vi "Controle_Manip_Main_GUI_Backup2.vi"() -> ()   [LabVIEW 2019] (continued)
                      tunnel: [w4532] -> w4511
                      tunnel: w4510 -> [w4531]
                      tunnel: w4509 -> [w4530]
                      frame #0 {
                        n3649 = call <instrlib>:"TL4000 Get LD Output State.vi"("error in (no error)"=w4516, "instrument handle"=w4523) -> ("error out"=w4518:errorcluster, "LD Output"=w4520:bool, "instrument handle out"=w4519:refnum<visa-resource-name>)  [unwired: 7 in]
                        n3650 = Not(x=w4520) -> (.not. x?=w4517:bool)
                        n3651 = case shown="True" w4517 {
                          selector: w4517 -> [w4525 w4526]
                          frame False {
                            n3652 = Not(x=w4525) -> (.not. x?=w4524:bool)
                            n3653 = property on="TEC Output" class="Bool (strict)"("Visible"=w4524) -> ()  [unwired: 2 in, 2 out]
                          }
                          frame True {
                            n3654 = property on="TEC Output" class="Bool (strict)"("Visible"=w4526) -> ()  [unwired: 2 in, 2 out]
                          }
                        }
                        n3655 = property on="Laser Diode Current Set" class="Slide (strict)"("Visible"=w4517) -> ()  [unwired: 2 in, 2 out]
                        n3656 = property on="Laser Safety" class="Ring (strict)"("Visible"=w4517) -> ()  [unwired: 2 in, 2 out]
                        n3657 = local write "Laser on?"(w4517) -> ()
                        n3658 = call <instrlib>:"TL4000 Switch LD Output.vi"("error in (no error)"=w4518, "LD Output (Off)"=w4517, "instrument handle"=w4519) -> ("error out"=w4522:errorcluster, "instrument handle out"=w4521:refnum<visa-resource-name>)  [unwired: 7 in]
                      }
                      frame #1 {
                        n3659 = local read "PM16-120 On?"() -> (w4527:bool)
                        n3660 = case shown="True" w4527 {
                          tunnel: [w4536 w4543] -> w4533
                          tunnel: [w4537 w4542] -> w4532
                          tunnel: w4531 -> [w4536 w4541]
                          tunnel: w4530 -> [w4537 w4540]
                          tunnel: [0.0 ("Power") w4539] -> w4529
                          frame False {
                          }
                          frame True {
                            n3661 = call <instrlib>:"TLPM Measure Power.vi"("error in (no error)"=w4540, "instrument handle"=w4541) -> ("error out"=w4542:errorcluster, "Power"=w4539:dbl, "instrument handle out"=w4543:refnum<visa-resource-name>)  [unwired: 7 in]
                          }
                        }
                        n3662 = local write "Excitation Power (uW)"(w4529) -> ()
                        n3663 = property on="Excitation Source" class="Enum (strict)"("Val(Sgnl)"=enum16{"P", "CW", "SK"}."CW" ("Value (Signaling)")) -> ()  [unwired: 2 in, 2 out]
                      }
                    }
                  }
                  frame "Laser Diode Current Set" {
                    n3664 = stacked-sequence {
                      seq-local: [w4556 _ _ _] -> [_ _ w4576 _]
                      seq-local: [w4555 _ _ _] -> [_ _ w4575 _]
                      tunnel: w4551 -> [w4560 _ _ _]
                      tunnel: w4544 -> [w4552 _ _ _]
                      tunnel: [_ _ w4576 _] -> w4550
                      tunnel: [_ _ w4575 _] -> w4545
                      tunnel: w4549 -> [_ _ w4574 _]
                      tunnel: w4548 -> [_ _ w4573 _]
                      tunnel: [_ _ w4572 _] -> w4547
                      tunnel: [_ _ w4571 _] -> w4546
                      frame #0 {
                        n3665 = local read "Laser Diode Current Set"() -> (w4553:dbl)
                        n3666 = call <instrlib>:"TL4000 Get Laser Diode Current Setpoint.vi"("error in (no error)"=w4552, "instrument handle"=w4560) -> ("error out"=w4557:errorcluster, "Laser Diode Current Setpoint"=w4559:dbl, "instrument handle out"=w4558:refnum<visa-resource-name>)  [unwired: 7 in]
                        n3667 = Not Equal?(x=w4553, y=w4559) -> (x != y?=w4554:bool)
                        n3668 = case shown="True" w4554 {
                          tunnel: w4558 -> [w4562 w4567]
                          tunnel: w4557 -> [w4561 w4566]
                          tunnel: [w4562 w4565] -> w4556
                          tunnel: [w4561 w4564] -> w4555
                          tunnel: w4553 -> [_ w4563]
                          frame False {
                          }
                          frame True {
                            n3669 = call <instrlib>:"TL4000 Set Laser Diode Current Setpoint.vi"("error in (no error)"=w4566, "Laser Diode Current Setpoint (0.0)"=w4563, "instrument handle"=w4567) -> ("error out"=w4564:errorcluster, "instrument handle out"=w4565:refnum<visa-resource-name>)  [unwired: 7 in]
                          }
                        }
                      }
                      frame #1 {
                        n3670 = Wait (ms)(milliseconds to wait=u32 50) -> ()  [unwired: 1 out]
                      }
                      frame #2 {
                        n3671 = local read "PM16-120 On?"() -> (w4569:bool)
                        n3672 = case shown="True" w4569 {
                          tunnel: w4574 -> [w4579 w4584]
                          tunnel: w4573 -> [w4578 w4583]
                          tunnel: [w4579 w4582] -> w4572
                          tunnel: [w4578 w4581] -> w4571
                          tunnel: [0.0 ("Power") w4580] -> w4570
                          frame False {
                          }
                          frame True {
                            n3673 = call <instrlib>:"TLPM Measure Power.vi"("error in (no error)"=w4583, "instrument handle"=w4584) -> ("error out"=w4581:errorcluster, "Power"=w4580:dbl, "instrument handle out"=w4582:refnum<visa-resource-name>)  [unwired: 7 in]
                          }
                        }
                        n3674 = local write "Excitation Power (uW)"(w4570) -> ()
                      }
                      frame #3 {
                        n3675 = local write "Background taken?"(FALSE ("Background taken?")) -> ()
                      }
                    }
                  }
                  frame "TEC Output" {
                    n3676 = local read "TEC Output"() -> (w4586:bool)
                    n3677 = call <instrlib>:"TL4000 Switch TEC Output.vi"("error in (no error)"=w4587, "TEC Output (Off)"=w4586, "instrument handle"=w4588) -> ("error out"=w4593:errorcluster, "instrument handle out"=w4594:refnum<visa-resource-name>)  [unwired: 7 in]
                    n3678 = case shown="True" w4586 {
                      tunnel: w4594 -> [w4596 w4603]
                      tunnel: w4593 -> [w4595 w4602]
                      tunnel: [w4596 w4599] -> w4590
                      tunnel: [w4595 w4598] -> w4589
                      frame False {
                      }
                      frame True {
                        n3679 = while {
                          tunnel: w4603 -> [w4617]
                          tunnel: [w4609] -> w4600
                          tunnel: w4602 -> [w4616]
                          tunnel: [w4610] -> w4601
                          stop <- w4604 stop-if-true
                          n3680 = call <instrlib>:"TL4000 Measure Temperature.vi"("error in (no error)"=w4616, "instrument handle"=w4617) -> ("error out"=w4610:errorcluster, "Temperature"=w4607:dbl, "instrument handle out"=w4609:refnum<visa-resource-name>)  [unwired: 7 in]
                          n3681 = Wait (ms)(milliseconds to wait=u32 250) -> ()  [unwired: 1 out]
                          n3682 = local write "TEC Temperature"(w4607) -> ()
                          n3683 = Subtract(x=w4607, y=25.0) -> (x-y=w4614:dbl)
                          n3684 = Absolute Value(x=w4614) -> (abs(x)=w4613:dbl)
                          n3685 = Equal?(x=w4607, y=0.0) -> (x = y?=w4605:bool)
                          n3686 = Less?(x=w4613, y=0.01) -> (x < y?=w4608:bool)
                          n3687 = Or(x=w4608, y=w4605) -> (x .or. y?=w4604:bool)
                        }
                        n3688 = call <instrlib>:"TL4000 Measure Temperature.vi"("error in (no error)"=w4601, "instrument handle"=w4600) -> ("error out"=w4598:errorcluster, "Temperature"=w4597:dbl, "instrument handle out"=w4599:refnum<visa-resource-name>)  [unwired: 7 in]
                        n3689 = local write "TEC Temperature"(w4597) -> ()
                      }
                    }
                    n3690 = property on="Laser on? Control" class="Bool (strict)"("Visible"=w4586) -> ()  [unwired: 2 in, 2 out]
                  }
                  frame Default {
                  }
                }
                "Diode Driver Error out" <- w4492
                n3691 = local write "Photodiode error out"(w4490) -> ()
                n3692 = local write "Photodiode handle out"(w4495) -> ()
                n3693 = local write "Diode Driver COM"(w4494) -> ()
              }
            }
          }
          event "Fit?": Mouse Down {
            n3694 = event-data() -> ()  [unwired: 1 in, 8 out]
            n3695 = property on="CCD 1D Spectrum Main" class="XYGraph (strict)"() -> ("Value"=w4626:cluster{dbl[], dbl[]})  [unwired: 2 in, 2 out]
            n3696 = local read "BackgroundSpec"() -> (w4622:dbl[])
            n3697 = Unbundle(w4626) -> (w4625:dbl[], w4623:dbl[])
            n3698 = call "subVI_FitLorentzien.vi"("Background Spec"=w4622, "X"=w4625, "Y"=w4623) -> ("best fit parameters"=→"best fit parameters":dbl[])  [unwired: 1 in, 3 out]
          }
          event "Temperature (K)": Mouse Down {
            n3699 = event-data() -> ()  [unwired: 1 in, 8 out]
            n3700 = local read "Cryostation On?"() -> (w4627:bool)
            n3701 = case shown="True" w4627 {
              frame False {
              }
              frame True {
                w4629 = 10.0 ("y")
                n3702 = local read "Cryostation ID"() -> (w4639:refnum<k5>)
                n3703 = call "GetCryoInfo.vi"("connection ID"=w4639) -> ("User Stability"=w4634:dbl, "User Temp"=w4635:dbl, "connection ID out"=w4633:refnum<k5>, "Sample Stability"=w4636:dbl, "Sample Temp"=w4632:dbl, "Platform Stability"=w4637:dbl, "Platform Temp"=w4638:dbl)  [unwired: 4 in]
                n3704 = local write "Cryo Platform Temp"(w4638) -> ()
                n3705 = Multiply(x=w4632, y=w4629) -> (x*y=w4631:dbl)
                n3706 = local write "Cryo Sample Stability"(w4636) -> ()
                n3707 = local write "Cryostation ID"(w4633) -> ()
                n3708 = local write "Cryo User Stability"(w4634) -> ()
                n3709 = local write "Cryo Sample Temp"(w4632) -> ()
                n3710 = local write "Cryo Platform Stability"(w4637) -> ()
                n3711 = local write "Cryo User Temp"(w4635) -> ()
                n3712 = Round To Nearest(number=w4631) -> (nearest integer value=w4630:dbl)
                n3713 = Divide(x=w4630, y=w4629) -> (x/y=w4628:dbl)
                n3714 = local write "Temperature (K)"(w4628) -> ()
              }
            }
          }
          event "Voltage Output?": Value Change {
            w4644 = u8 2 items=["1", "2", "3"] ("axis")
            w4645 = u8 1 items=["1", "2", "3"] ("axis")
            w4646 = u8 0 items=["1", "2", "3"] ("axis")
            n3715 = event-data() -> ("NewVal"=w4640:bool)  [unwired: 1 in, 5 out]
            n3716 = local read "Att Error"() -> (w4653:errorcluster)
            n3717 = local read "Att DeviceHandle"() -> (w4655:u64)
            n3718 = local read "ourDLL"() -> (w4643:path)
            n3719 = call "ANC350v4_SetAxisOutput.vi"("deviceHandle"=w4655, "Path to *.DLL"=w4643, "axis"=w4646, "enable"=w4640, "autoDisable"=TRUE, "error in"=w4653) -> ("deviceHandle"=w4651:u64, "error ANC350v4_setAxisOutput"=w4652:errorcluster)  [unwired: 7 in, 1 out]
            n3720 = call "ANC350v4_SetAxisOutput.vi"("deviceHandle"=w4651, "Path to *.DLL"=w4643, "axis"=w4645, "enable"=w4640, "autoDisable"=TRUE, "error in"=w4652) -> ("deviceHandle"=w4650:u64, "error ANC350v4_setAxisOutput"=w4649:errorcluster)  [unwired: 7 in, 1 out]
            n3721 = call "ANC350v4_SetAxisOutput.vi"("deviceHandle"=w4650, "Path to *.DLL"=w4643, "axis"=w4644, "enable"=w4640, "autoDisable"=TRUE, "error in"=w4649) -> ("deviceHandle"=w4642:u64, "error ANC350v4_setAxisOutput"=w4641:errorcluster)  [unwired: 7 in, 1 out]
            n3722 = local write "Att Error"(w4641) -> ()
            n3723 = local write "Att DeviceHandle"(w4642) -> ()
          }
          event Timeout {
            # "Use timeout case to send data to globals"
            n3724 = event-data() -> ()  [unwired: 1 in, 3 out]
          }
        }
      }
      n3725 = while {
        stop <- w723 stop-if-true
        # "Separate loop for \"measurements\" requiring simultaneous optimisation of experimental parameters"
        n3726 = event shown="[2] \"Acquire PD\": Mouse Down" {
          selector: _ -> [_ _ _]
          dyn-events: _ -> [_ _ _]
          timeout: 500 -> [_ _ _]
          event Timeout {
            n3727 = event-data() -> ()  [unwired: 1 in, 3 out]
          }
          event "Fast Acq Continuous": Mouse Down {
            n3728 = event-data() -> ()  [unwired: 1 in, 8 out]
            n3729 = local read "Acq Mode"() -> (w724:T3)
            n3730 = case shown="\"Spectrum\", Default" w724 {
              frame "Image" {
              }
              frame "APD 1" {
              }
              frame "Spectrum", Default {
                n3731 = stacked-sequence {
                  frame #0 {
                    # "prep stuff"
                    n3732 = property on="Experiment Graph Controls" class="TabCtl (strict)"("Value"=T25."Spectrum" ("Experiment Graph Controls")) -> ()  [unwired: 2 in, 2 out]
                  }
                  frame #1 {
                    # "open shutter once"
                    n3733 = control-ref of="Shutter Ctrls"() -> (w731:refnum<vi>)
                    n3734 = local read "KCube Shutter On?"() -> (w728:bool)
                    n3735 = local read "Acq Mode"() -> (w729:T3)
                    n3736 = control-ref of="KCube Shutter Device Reference"() -> (w730:refnum<vi>)
                    n3737 = call "Shutter.vi"("KCube Shutter Device Reference 2"=w730, "Shutter Ctrls 2"=w731, "Shutter on?"=w728) -> ()
                    n3738 = case shown="\"Spectrum\", Default" w729 {
                      frame "Spectrum", Default {
                        n3739 = property on="CCD 1D Spectrum Main" class="XYGraph (strict)"("Visible"=TRUE) -> ()  [unwired: 2 in, 2 out]
                        n3740 = property on="CCD 2D Image Main" class="IntGraph (strict)"("Visible"=FALSE) -> ()  [unwired: 2 in, 2 out]
                      }
                      frame "Image" {
                        n3741 = property on="CCD 1D Spectrum Main" class="XYGraph (strict)"("Visible"=FALSE) -> ()  [unwired: 2 in, 2 out]
                        n3742 = property on="CCD 2D Image Main" class="IntGraph (strict)"("Visible"=TRUE) -> ()  [unwired: 2 in, 2 out]
                      }
                    }
                    n3743 = control-ref of="MasterStop"() -> (w727:refnum<vi>)
                    n3744 = property class="Bool (strict)"(reference=w727, "Visible"=TRUE) -> ()  [unwired: 1 in, 2 out]
                  }
                  frame #2 {
                    # "acquire 1000 spectra"
                    n3745 = for {
                      N: 1000 -> [_]
                      stop <- w751 stop-if-true
                      n3746 = local read "CCD ROI"() -> (w746:T20)
                      n3747 = local read "LightField Automation out"() -> (w750:refnum<class "LightField Automation.lvclass">)
                      n3748 = local read "Acq Mode"() -> (w753:T3)
                      n3749 = local read "LightField Automation error out"() -> (w747:errorcluster)
                      n3750 = local read "Accumulations"() -> (w754:dbl)
                      n3751 = control-ref of="MasterStop"() -> (w737:refnum<vi>)
                      n3752 = local read "BackgroundSpec"() -> (w739:dbl[])
                      n3753 = local read "Excitation Power (uW)"() -> (w742:dbl)
                      n3754 = call "LFA_Capture.vi"("error in (no error)"=w747, "Frames"=w754, "LightField Automation in"=w750) -> ("error out"=w748:errorcluster, "Data"=w752:T26, "LightField Automation out"=w749:refnum<class "LightField Automation.lvclass">)  [unwired: 6 in]
                      n3755 = case shown="\"Spectrum\", Default" w753 {
                        selector: w753 -> [w762 w768]
                        tunnel: w752 -> [w763 w770]
                        tunnel: w746 -> [w759 w765]
                        tunnel: [w755 w764] -> w743
                        frame "Spectrum", Default {
                          n3756 = local read "Wavelength calibration"() -> (w757:dbl[])
                          n3757 = Divide(x=1239.842, y=w757) -> (x/y=w756:dbl[])
                          n3758 = call "PrepareData4Graph.vi"("Wavelength nm"=w756, "DataLF"=w763, "CCD ROI"=w759, "AcqMode"=w762, "Data type"=T30."Spectre") -> ("Spectrum"=w761:cluster{"Array 2":dbl[], "Array":dbl[]}, "PLInt out"=w755:dbl[])  [unwired: 2 in, 2 out]
                          n3759 = local write "CCD 1D Spectrum Main"(w761) -> ()
                        }
                        frame "Image" {
                          n3760 = local read "Wavelength calibration"() -> (w769:dbl[])
                          n3761 = call "PrepareData4Graph.vi"("Wavelength nm"=w769, "DataLF"=w770, "CCD ROI"=w765, "AcqMode"=w768, "Data type"=T30."Spectre") -> ("Intensity Graph"=w767:dbl[][], "PLInt out"=w764:dbl[])  [unwired: 2 in, 2 out]
                          n3762 = local write "CCD 2D Image Main"(w767) -> ()
                        }
                      }
                      n3763 = call "myMax.vi"("Array"=w743) -> ("myMax"=w745:dbl)  [unwired: 1 in]
                      n3764 = property on="CCD 1D Spectrum Main" class="XYGraph (strict)"("YScale.Maximum"=w745, "YScale.Minimum"=0.0 ("Y Scale.Range:Minimum")) -> ()  [unwired: 2 in, 2 out]
                      n3765 = local read "Acq Time (ms)"() -> (w741:dbl)
                      n3766 = local read "Display Mode"() -> (w738:u16)
                      n3767 = local write "LightField Automation out"(w749) -> ()
                      n3768 = local write "LightField Automation error out"(w748) -> ()
                      n3769 = property class="Bool (strict)"(reference=w737) -> ("Value"=w751:bool)  [unwired: 1 in, 2 out]
                      n3770 = control-ref of="Cnts"() -> (w740:refnum<vi>)
                      n3771 = call "2Cnts.vi"("Array Background"=w739, "Pow W"=w742, "AcqTime ms"=w741, "Cnts Ref"=w740, "Display Mode"=w738, "Array"=w743) -> ()  [unwired: 1 out]
                    }
                  }
                  frame #3 {
                    # "close shutter"
                    n3772 = local read "KCube Shutter On?"() -> (w774:bool)
                    n3773 = control-ref of="Fast Acq Continuous"() -> (w772:refnum<vi>)
                    n3774 = control-ref of="Shutter Ctrls"() -> (w778:refnum<vi>)
                    n3775 = control-ref of="KCube Shutter Device Reference"() -> (w777:refnum<vi>)
                    n3776 = control-ref of="MasterStop"() -> (w773:refnum<vi>)
                    n3777 = property class="Bool (strict)"(reference=w772, "Value"=FALSE) -> ()  [unwired: 1 in, 2 out]
                    n3778 = call "Shutter.vi"("KCube Shutter Device Reference 2"=w777, "Shutter Ctrls 2"=w778, "Shutter on?"=w774) -> ()
                    n3779 = property class="Bool (strict)"(reference=w773, "Value"=FALSE, "Visible"=FALSE) -> ()  [unwired: 1 in, 2 out]
                  }
                }
              }
            }
          }
          event "Acquire PD": Mouse Down {
            n3780 = event-data() -> ()  [unwired: 1 in, 8 out]
            n3781 = local read "PicoHarp On?"() -> (w779:bool)
            n3782 = case shown="True" w779 {
              frame False {
              }
              frame True {
                n3783 = local read "Spectrum Custom Continuous Mode"() -> (w780:u16)
                n3784 = case shown="3" w780 {
                  frame 0, Default {
                    # "PD 2"
                    n3785 = stacked-sequence {
                      frame #0 {
                        n3786 = property on="Experiment Graph Controls" class="TabCtl (strict)"("Value"=T25."APDs" ("Experiment Graph Controls")) -> ()  [unwired: 2 in, 2 out]
                      }
                      frame #1 {
                        n3787 = for {
                          N: 1000 -> [_]
                          shift-right: [w786] -> _
                          shift-left: dbl[] [] -> [w791]
                          stop <- w784 stop-if-true
                          n3788 = local read "Photodiode handle out"() -> (w797:refnum<visa-resource-name>)
                          n3789 = local read "Photodiode error out"() -> (w796:errorcluster)
                          n3790 = control-ref of="PD 1D Spectrum"() -> (w788:refnum<vi>)
                          n3791 = Tick Count (ms)() -> (millisecond timer value=w793:u32)
                          n3792 = while {
                            shift-right: [w807] -> w795
                            shift-left: w797 -> [w810]
                            shift-right: [w806] -> w794
                            shift-left: w796 -> [w809]
                            tunnel: w793 -> [w803]
                            shift-right: [w798] -> w790
                            shift-left: dbl[] [] -> [w800]
                            stop <- w802 stop-if-true
                            n3793 = local read "Acq Time (ms)"() -> (w801:dbl)
                            n3794 = Tick Count (ms)() -> (millisecond timer value=w805:u32)
                            n3795 = call <instrlib>:"TLPM Measure Power.vi"("error in (no error)"=w809, "instrument handle"=w810) -> ("error out"=w806:errorcluster, "Power"=w799:dbl, "instrument handle out"=w807:refnum<visa-resource-name>)  [unwired: 7 in]
                            n3796 = control-ref of="Excitation Power (uW)"() -> (w808:refnum<vi>)
                            n3797 = property class="DigNum (strict)"(reference=w808, "Value"=w799) -> ()  [unwired: 1 in, 2 out]
                            n3798 = Subtract(x=w805, y=w803) -> (x-y=w804:u32)
                            n3799 = Insert Into Array(array=w800, new element=w799) -> (w798:dbl[])  [unwired: 1 in]
                            n3800 = Greater?(x=w804, y=w801) -> (0:w802:bool)
                          }
                          n3801 = control-ref of="Stop PD"() -> (w785:refnum<vi>)
                          n3802 = local write "Photodiode handle out"(w795) -> ()
                          n3803 = call-poly <vilib>:"Mean.vi"("X"=w790) -> ("mean"=w789:dbl)  [unwired: 1 out]
                          n3804 = Insert Into Array(array=w791, new element=w789) -> (w786:dbl[])  [unwired: 1 in]
                          n3805 = Build Array(w786) -> (w787:dbl[][])
                          n3806 = property class="WFGraph (strict)"(reference=w788, "Value"=w787) -> ()  [unwired: 1 in, 2 out]
                          n3807 = local write "Photodiode error out"(w794) -> ()
                          n3808 = property class="Bool (strict)"(reference=w785) -> ("Value"=w784:bool)  [unwired: 1 in, 2 out]
                        }
                      }
                      frame #2 {
                        w811 = FALSE ("Stop PD")
                        n3809 = property on="Acquire PD" class="Bool (strict)"("Value"=w811) -> ()  [unwired: 2 in, 2 out]
                        n3810 = property on="Stop PD" class="Bool (strict)"("Value"=w811) -> ()  [unwired: 2 in, 2 out]
                      }
                    }
                  }
                  frame 3 {
                    # "APD1+2"
                    n3811 = stacked-sequence {
                      frame #0 {
                        n3812 = local read "PH_Init_Data"() -> (w824:T11)
                        n3813 = Unbundle By Name(w824) -> ("Deviceindex"=w816:i32)
                        n3814 = local read "PH_Settings_Params"() -> (w817:T10)
                        n3815 = local read "PH_CFD1 level"() -> (w821:i32)
                        n3816 = local read "PH_CFD1 zero X"() -> (w820:i32)
                        n3817 = local read "Acq Time (ms)"() -> (w819:dbl)
                        n3818 = local read "PH_Range No."() -> (w815:i32)
                        n3819 = local read "PH_CFD0 level"() -> (w822:i32)
                        n3820 = local read "PH_CFD0 zero X"() -> (w814:i32)
                        n3821 = local read "PH_SyncDiv"() -> (w823:enum16{"1", "2", "4", "8"})
                        n3822 = property on="Experiment Graph Controls" class="TabCtl (strict)"("Value"=T25."APDs" ("Experiment Graph Controls")) -> ()  [unwired: 2 in, 2 out]
                        n3823 = Bundle By Name(cluster=w817, "SyncDiv"=w823, "DeviceIndex"=w816, "CFD0 level"=w822, "CFD0 zero X"=w814, "CFD1 level"=w821, "CFD1 zero X"=w820, "Range No."=w815, "StopOnOverflow"=TRUE, "AcqTime (ms)"=w819) -> (w812:T10)
                        n3824 = local write "PH_Settings_Params"(w812) -> ()
                      }
                      frame #1 {
                        n3825 = local read "PH_Init_Data"() -> (w827:T11)
                        n3826 = local read "PH_Settings_Params"() -> (w828:T10)
                        n3827 = control-ref of="Stop PD"() -> (w829:refnum<vi>)
                        n3828 = control-ref of="PD 1D Spectrum"() -> (w830:refnum<vi>)
                        n3829 = call "PH_GetRates_SubVI.vi"("APD num"=enum16{"NA", "APD1", "APD2", "APD1+2"}."APD1+2", "PH_Settings_Params"=w828, "PH_Init_Data"=w827, "Stop PD Ref"=w829, "PD 1D Spectrum Ref"=w830) -> ("APD1+2"=w825:dbl[][])  [unwired: 6 in]
                        n3830 = local write "PD Data 2D 2"(w825) -> ()
                      }
                      frame #2 {
                        w831 = FALSE ("Stop PD")
                        n3831 = property on="Acquire PD" class="Bool (strict)"("Value"=w831) -> ()  [unwired: 2 in, 2 out]
                        n3832 = property on="Stop PD" class="Bool (strict)"("Value"=w831) -> ()  [unwired: 2 in, 2 out]
                      }
                    }
                  }
                  frame 1 {
                    # "APD1"
                    n3833 = stacked-sequence {
                      frame #0 {
                        n3834 = local read "PH_Init_Data"() -> (w844:T11)
                        n3835 = Unbundle By Name(w844) -> ("Deviceindex"=w836:i32)
                        n3836 = local read "PH_Settings_Params"() -> (w837:T10)
                        n3837 = local read "PH_CFD1 level"() -> (w841:i32)
                        n3838 = local read "PH_CFD1 zero X"() -> (w840:i32)
                        n3839 = local read "Acq Time (ms)"() -> (w839:dbl)
                        n3840 = local read "PH_Range No."() -> (w835:i32)
                        n3841 = local read "PH_CFD0 level"() -> (w842:i32)
                        n3842 = local read "PH_CFD0 zero X"() -> (w834:i32)
                        n3843 = local read "PH_SyncDiv"() -> (w843:enum16{"1", "2", "4", "8"})
                        n3844 = property on="Experiment Graph Controls" class="TabCtl (strict)"("Value"=T25."APDs" ("Experiment Graph Controls")) -> ()  [unwired: 2 in, 2 out]
                        n3845 = Bundle By Name(cluster=w837, "SyncDiv"=w843, "DeviceIndex"=w836, "CFD0 level"=w842, "CFD0 zero X"=w834, "CFD1 level"=w841, "CFD1 zero X"=w840, "Range No."=w835, "StopOnOverflow"=TRUE, "AcqTime (ms)"=w839) -> (w832:T10)
                        n3846 = local write "PH_Settings_Params"(w832) -> ()
                      }
                      frame #1 {
                        n3847 = local read "PH_Init_Data"() -> (w847:T11)
                        n3848 = local read "PH_Settings_Params"() -> (w848:T10)
                        n3849 = control-ref of="Stop PD"() -> (w849:refnum<vi>)
                        n3850 = control-ref of="PD 1D Spectrum"() -> (w850:refnum<vi>)
                        n3851 = call "PH_GetRates_SubVI.vi"("APD num"=enum16{"NA", "APD1", "APD2", "APD1+2"}."APD1", "PH_Settings_Params"=w848, "PH_Init_Data"=w847, "Stop PD Ref"=w849, "PD 1D Spectrum Ref"=w850) -> ("APD1+2"=w845:dbl[][])  [unwired: 6 in]
                        n3852 = local write "PD Data 2D 2"(w845) -> ()
                      }
                      frame #2 {
                        w851 = FALSE ("Stop PD")
                        n3853 = property on="Acquire PD" class="Bool (strict)"("Value"=w851) -> ()  [unwired: 2 in, 2 out]
                        n3854 = property on="Stop PD" class="Bool (strict)"("Value"=w851) -> ()  [unwired: 2 in, 2 out]
                      }
                    }
                  }
                  frame 2 {
                    # "APD2"
                    n3855 = stacked-sequence {
                      frame #0 {
                        n3856 = local read "PH_Init_Data"() -> (w864:T11)
                        n3857 = Unbundle By Name(w864) -> ("Deviceindex"=w856:i32)
                        n3858 = local read "PH_Settings_Params"() -> (w857:T10)
                        n3859 = local read "PH_CFD1 level"() -> (w861:i32)
                        n3860 = local read "PH_CFD1 zero X"() -> (w860:i32)
                        n3861 = local read "Acq Time (ms)"() -> (w859:dbl)
                        n3862 = local read "PH_Range No."() -> (w855:i32)
                        n3863 = local read "PH_CFD0 level"() -> (w862:i32)
                        n3864 = local read "PH_CFD0 zero X"() -> (w854:i32)
                        n3865 = local read "PH_SyncDiv"() -> (w863:enum16{"1", "2", "4", "8"})
                        n3866 = property on="Experiment Graph Controls" class="TabCtl (strict)"("Value"=T25."APDs" ("Experiment Graph Controls")) -> ()  [unwired: 2 in, 2 out]
                        n3867 = Bundle By Name(cluster=w857, "SyncDiv"=w863, "DeviceIndex"=w856, "CFD0 level"=w862, "CFD0 zero X"=w854, "CFD1 level"=w861, "CFD1 zero X"=w860, "Range No."=w855, "StopOnOverflow"=TRUE, "AcqTime (ms)"=w859) -> (w852:T10)
                        n3868 = local write "PH_Settings_Params"(w852) -> ()
                      }
                      frame #1 {
                        n3869 = local read "PH_Init_Data"() -> (w867:T11)
                        n3870 = local read "PH_Settings_Params"() -> (w868:T10)
                        n3871 = control-ref of="Stop PD"() -> (w869:refnum<vi>)
                        n3872 = control-ref of="PD 1D Spectrum"() -> (w870:refnum<vi>)
                        n3873 = call "PH_GetRates_SubVI.vi"("APD num"=enum16{"NA", "APD1", "APD2", "APD1+2"}."APD2", "PH_Settings_Params"=w868, "PH_Init_Data"=w867, "Stop PD Ref"=w869, "PD 1D Spectrum Ref"=w870) -> ("APD1+2"=w865:dbl[][])  [unwired: 6 in]
                        n3874 = local write "PD Data 2D 2"(w865) -> ()
                      }
                      frame #2 {
                        w871 = FALSE ("Stop PD")
                        n3875 = property on="Acquire PD" class="Bool (strict)"("Value"=w871) -> ()  [unwired: 2 in, 2 out]
                        n3876 = property on="Stop PD" class="Bool (strict)"("Value"=w871) -> ()  [unwired: 2 in, 2 out]
                      }
                    }
                  }
                }
              }
            }
          }
        }
        n3877 = local read "NewVal"() -> (w723:bool)
      }
    }
    frame #3 {
      # "Shutdown: close all open references and connections"
      n3878 = stacked-sequence {
        frame #0 {
          # "Is the sample to be kept and reused?\ni.e. does LabVIEW keep sample details or empty them"
          n3879 = Two Button Dialog(message="Do you want to keep the sample details in LV?", 1:"No thanks." ("F button name (\"Cancel\")"), 2:"Yes please!" ("T button name (\"OK\")")) -> (T button?=w4656:bool)
          n3880 = case shown="False" w4656 {
            frame False {
              n3881 = local write "SampleGoal"("") -> ()
            }
            frame True {
            }
          }
        }
        frame #1 {
          # "Shutdown all connections"
          n3882 = local read "Initialise all devices?"() -> (w4661:bool)
          n3883 = case shown="True" w4661 {
            frame False {
              # "No devices to deactivate"
            }
            frame True {
              # "Deactivate all the selected devices"
              n3884 = stacked-sequence {
                frame #0 {
                  # "Message to user"
                  n3885 = local read "Log file"() -> (w4665:string)
                  n3886 = call "Write2LogFile.vi"("Add to log file"="Closing all connections ...", "Log file before"=w4665, "Checkbox"=FALSE) -> ("Log file after"=w4664:string)
                  n3887 = local write "Log file"(w4664) -> ()
                }
                frame #1 {
                  # "LLTF"
                  n3888 = local read "LLTF On?"() -> (w4666:bool)
                  n3889 = case shown="True" w4666 {
                    frame False {
                    }
                    frame True {
                      n3890 = local read "LLTF Reference"() -> (w4668:refnum<k7>)
                      n3891 = local read "LLTF Error"() -> (w4667:errorcluster)
                      n3892 = Close Reference(reference=w4668, error in (no error)=w4667) -> ()  [unwired: 1 out]
                    }
                  }
                }
                frame #2 {
                  # "turn off laser output, TEC and close connection"
                  # "448.3nm Laser Diode + Temp Controller & Driver"
                  n3893 = local read "Laser Comm On?"() -> (w4669:bool)
                  n3894 = case shown="True" w4669 {
                    frame False {
                      w4670 = TRUE ("Visible")
                      n3895 = property on="TEC Output" class="Bool (strict)"("Visible"=w4670) -> ()  [unwired: 2 in, 2 out]
                      n3896 = property on="TEC Temperature" class="DigNum (strict)"("Visible"=w4670) -> ()  [unwired: 2 in, 2 out]
                    }
                    frame True {
                      w4672 = FALSE ("TEC Output (Off)")
                      w4671 = FALSE ("LD Output (Off)")
                      # "laser"
                      n3897 = local read "Diode Driver COM"() -> (w4674:refnum<visa-resource-name>)
                      n3898 = local read "Diode Driver Error"() -> (w4673:errorcluster)
                      n3899 = property on="Laser on? Control" class="Bool (strict)"("Visible"=w4671) -> ()  [unwired: 2 in, 2 out]
                      n3900 = Not(x=w4671) -> (.not. x?=w4679:bool)
                      n3901 = call <instrlib>:"TL4000 Switch LD Output.vi"("error in (no error)"=w4673, "LD Output (Off)"=w4671, "instrument handle"=w4674) -> ("error out"=w4675:errorcluster, "instrument handle out"=w4678:refnum<visa-resource-name>)  [unwired: 7 in]
                      n3902 = property on="Laser Safety" class="Ring (strict)"("Visible"=w4671) -> ()  [unwired: 2 in, 2 out]
                      n3903 = local write "Laser on?"(w4671) -> ()
                      n3904 = local write "Laser on? Control"(w4671) -> ()
                      n3905 = property on="TEC Output" class="Bool (strict)"("Visible"=w4679) -> ()  [unwired: 2 in, 2 out]
                      n3906 = call <instrlib>:"TL4000 Switch TEC Output.vi"("error in (no error)"=w4675, "TEC Output (Off)"=w4672, "instrument handle"=w4678) -> ("error out"=w4676:errorcluster, "instrument handle out"=w4677:refnum<visa-resource-name>)  [unwired: 7 in]
                      n3907 = call <instrlib>:"TL4000 Close.vi"("error in (no error)"=w4676, "instrument handle"=w4677) -> ()  [unwired: 9 in, 1 out]
                      n3908 = local write "TEC Output"(w4672) -> ()
                      n3909 = property on="Laser Diode Current Set" class="Slide (strict)"("Visible"=w4671) -> ()  [unwired: 2 in, 2 out]
                      n3910 = property on="TEC Temperature" class="DigNum (strict)"("Visible"=w4679) -> ()  [unwired: 2 in, 2 out]
                    }
                  }
                }
                frame #3 {
                  # "KCubes: 1 Shutter + 3 Piezos"
                  n3911 = local read "KCubes Piezo On?"() -> (w4681:bool)
                  n3912 = case shown="True" w4681 {
                    frame False {
                    }
                    frame True {
                      # "Close piezo controls and shutter device"
                      n3913 = local read "KCubePiezoControl Y Reference"() -> (w4684:refnum<k24>)
                      n3914 = local read "KCubePiezoControl X Reference"() -> (w4683:refnum<k24>)
                      n3915 = local read "KCubePiezoControl Z Reference"() -> (w4685:refnum<k24>)
                      n3916 = invoke class="KCubePiezoControl" method="CloseDevice"(reference=w4684) -> ()  [unwired: 2 in, 3 out]
                      n3917 = invoke class="KCubePiezoControl" method="CloseDevice"(reference=w4683) -> ()  [unwired: 2 in, 3 out]
                      n3918 = invoke class="KCubePiezoControl" method="CloseDevice"(reference=w4685) -> ()  [unwired: 2 in, 3 out]
                    }
                  }
                  n3919 = local read "KCube Shutter On?"() -> (w4680:bool)
                  n3920 = case shown="True" w4680 {
                    frame False {
                    }
                    frame True {
                      n3921 = local read "KCubeSolenoidControl Reference"() -> (w4682:refnum<k24>)
                      n3922 = invoke class="KCubeSolenoidControl" method="CloseDevice"(reference=w4682) -> ()  [unwired: 2 in, 3 out]
                    }
                  }
                }
                frame #4 {
                  # "LightField: SpectraPro Mono + CCD"
                  n3923 = local read "LightField On?"() -> (w4686:bool)
                  n3924 = case shown="True" w4686 {
                    frame False {
                    }
                    frame True {
                      n3925 = local read "LightField Automation error out"() -> (w4687:errorcluster)
                      n3926 = local read "LightField Automation out"() -> (w4688:refnum<class "LightField Automation.lvclass">)
                      n3927 = call "LFA_Close.vi"("error in (no error)"=w4687, "LightField Automation in"=w4688) -> ()  [unwired: 8 in, 2 out]
                    }
                  }
                }
                frame #5 {
                  # "ESP 301: 2 rotation stages + 1 linear translation stage"
                  n3928 = local read "ESP 301 On?"() -> (w4689:bool)
                  n3929 = case shown="True" w4689 {
                    frame False {
                    }
                    frame True {
                      n3930 = local read "ESP 301 COM Port"() -> (w4690:refnum<visa-resource-name>)
                      n3931 = call "Close.vi"("VISA resource name"=w4690) -> ()  [unwired: 10 in, 1 out]
                    }
                  }
                }
                frame #6 {
                  # "ESP 300: Mono Jobin Yvon"
                  n3932 = local read "ESP 300 On?"() -> (w4691:bool)
                  n3933 = case shown="True" w4691 {
                    frame False {
                    }
                    frame True {
                      n3934 = local read "ESP300 COM Port"() -> (w4692:refnum<visa-resource-name>)
                      n3935 = local read "ESP300 Error"() -> (w4693:errorcluster)
                      n3936 = call "Uninit Communication.vi"("error in (no error)"=w4693, "VISA resource name in"=w4692) -> ()  [unwired: 9 in, 1 out]
                    }
                  }
                }
                frame #7 {
                  # "Thorlabs USB photodiode"
                  n3937 = local read "PM16-120 On?"() -> (w4694:bool)
                  n3938 = case shown="True" w4694 {
                    frame False {
                    }
                    frame True {
                      # "photo"
                      n3939 = local read "Photodiode error out"() -> (w4699:errorcluster)
                      n3940 = call <instrlib>:"TLPM Measure Power.vi"("error in (no error)"=w4699, "instrument handle"=refnum<visa-resource-name> "USB0::0x1313::0x807B::190927109::INSTR") -> ("error out"=w4697:errorcluster, "Power"=w4696:dbl, "instrument handle out"=w4698:refnum<visa-resource-name>)  [unwired: 7 in]
                      n3941 = call <instrlib>:"TLPM Close.vi"("error in (no error)"=w4697, "instrument handle"=w4698) -> ("error out"=w4700:errorcluster)  [unwired: 9 in]
                      n3942 = local write "Excitation Power (uW)"(w4696) -> ()
                      n3943 = local write "Photodiode error out"(w4700) -> ()
                    }
                  }
                }
                frame #8 {
                  # "Attocubes disconnect"
                  n3944 = local read "Attocubes On?"() -> (w4701:bool)
                  n3945 = case shown="True" w4701 {
                    frame False {
                    }
                    frame True {
                      w4707 = u8 2 items=["1", "2", "3"] ("axis")
                      w4708 = u8 1 items=["1", "2", "3"] ("axis")
                      w4717 = u8 0 items=["1", "2", "3"] ("axis")
                      w4706 = FALSE ("ANC connected")
                      n3946 = local read "Att DeviceHandle"() -> (w4719:u64)
                      n3947 = local read "Att Error"() -> (w4718:errorcluster)
                      n3948 = local read "ourDLL"() -> (w4705:path)
                      n3949 = call "ANC350v4_SetAxisOutput.vi"("deviceHandle"=w4719, "Path to *.DLL"=w4705, "axis"=w4717, "enable"=FALSE, "autoDisable"=TRUE, "error in"=w4718) -> ("deviceHandle"=w4711:u64, "error ANC350v4_setAxisOutput"=w4716:errorcluster)  [unwired: 7 in, 1 out]
                      n3950 = call "ANC350v4_SetAxisOutput.vi"("deviceHandle"=w4711, "Path to *.DLL"=w4705, "axis"=w4708, "enable"=FALSE, "autoDisable"=TRUE, "error in"=w4716) -> ("deviceHandle"=w4712:u64, "error ANC350v4_setAxisOutput"=w4715:errorcluster)  [unwired: 7 in, 1 out]
                      n3951 = call "ANC350v4_SetAxisOutput.vi"("deviceHandle"=w4712, "Path to *.DLL"=w4705, "axis"=w4707, "enable"=FALSE, "autoDisable"=TRUE, "error in"=w4715) -> ("deviceHandle"=w4713:u64, "error ANC350v4_setAxisOutput"=w4714:errorcluster)  [unwired: 7 in, 1 out]
                      n3952 = call "ANC350v4sub_Disconnect.vi"("ANC350v4_Handle"=w4713, "Path to *.DLL"=w4705, "error in"=w4714) -> ("error ANC350v4_Dis/Connect"=w4721:errorcluster)  [unwired: 12 in]
                      n3953 = local write "Voltage Output?"(w4706) -> ()
                      n3954 = local write "ANC connected"(w4706) -> ()
                      n3955 = local write "Att Error"(w4721) -> ()
                    }
                  }
                }
                frame #9 {
                  # "Montana Cryostation s50"
                  n3956 = local read "Cryostation On?"() -> (w4722:bool)
                  n3957 = case shown="True" w4722 {
                    frame False {
                    }
                    frame True {
                      n3958 = local read "Cryostation ID"() -> (w4723:refnum<k5>)
                      n3959 = call "CryoDisconnect.vi"("connection ID"=w4723) -> ()
                    }
                  }
                }
                frame #10 {
                  n3960 = local read "PicoHarp On?"() -> (w4724:bool)
                  n3961 = case shown="True" w4724 {
                    frame False {
                    }
                    frame True {
                      n3962 = local read "PH_Init_Data"() -> (w4727:T11)
                      n3963 = Unbundle By Name(w4727) -> ("Deviceindex"=w4726:i32)
                      n3964 = local write "Connected"(FALSE) -> ()
                      n3965 = call "PH_Close.vi"("devidx"=w4726) -> ()
                    }
                  }
                }
              }
            }
          }
        }
        frame #2 {
          # "Save log file & empty strings for next operation"
          n3966 = local read "Initialise all devices?"() -> (w4728:bool)
          n3967 = property on="Experiment Graph Controls" class="TabCtl (strict)"() -> ("Pages"=w4733:refnum<vi>[])  [unwired: 2 in, 2 out]
          n3968 = case shown="True" w4728 {
            frame False {
            }
            frame True {
              n3969 = stacked-sequence {
                frame #0 {
                  # "save log file"
                  n3970 = local read "Experiment Name"() -> (w4736:string)
                  n3971 = local read "Log file"() -> (w4737:string)
                  n3972 = call "CreatePath.vi"("filetype"=enum16{".h5", ".txt"}.".txt", "FileName"=w4736) -> ("File path"=w4734:path)
                  n3973 = Write to Text File(file (use dialog)=w4734, text=w4737) -> ()  [unwired: 2 in, 3 out]
                }
              }
            }
          }
          n3974 = Index Array(array=w4733, index=6) -> (element=w4731:refnum<vi>)
          n3975 = property class="Page"(reference=w4731, "PageVis"=TRUE ("Page Visible")) -> ()  [unwired: 1 in, 2 out]
          n3976 = property on="Experiment Graph Controls" class="TabCtl (strict)"("Value"=T25."Settings" ("Experiment Graph Controls")) -> ()  [unwired: 2 in, 2 out]
        }
      }
    }
  }
  n3977 = disable-structure shown="Disabled" {
    frame Disabled {
      n3978 = stacked-sequence {
        tunnel: [_ _ w4786] -> w4739
        frame #0 {
          n3979 = property on="CCD 1D Spectrum Main" class="XYGraph (strict)"("YScale.Offset"=0.0 ("Y Scale.Offset and Multiplier:Offset")) -> ()  [unwired: 2 in, 2 out]
          n3980 = local read "Log file"() -> (w4771:string)
          n3981 = call "Write2LogFile.vi"("Add to log file"="Acquiring background", "Log file before"=w4771) -> ("Log file after"=w4770:string)
          n3982 = local write "Log file"(w4770) -> ()
        }
        frame #1 {
          # "make sure shutter is closed"
          n3983 = control-ref of="Shutter Ctrls"() -> (w4776:refnum<vi>)
          n3984 = control-ref of="KCube Shutter Device Reference"() -> (w4777:refnum<vi>)
          n3985 = property class="Ring (strict)"(reference=w4776) -> ("Value"=w4775:u16)  [unwired: 1 in, 2 out]
          n3986 = local read "KCube Shutter On?"() -> (w4772:bool)
          n3987 = Equal?(x=w4775, y=u16 0) -> (x = y?=w4773:bool)
          n3988 = case shown="False" w4773 {
            tunnel: w4777 -> [w4780 _]
            tunnel: w4776 -> [w4779 _]
            tunnel: w4772 -> [w4778 _]
            frame False {
              n3989 = call "Shutter.vi"("KCube Shutter Device Reference 2"=w4780, "Shutter Ctrls 2"=w4779, "Shutter on?"=w4778) -> ()
            }
            frame True {
            }
          }
        }
        frame #2 {
          # "acquire"
          n3990 = local read "LightField Automation error out"() -> (w4784:errorcluster)
          n3991 = local read "LightField Automation out"() -> (w4785:refnum<class "LightField Automation.lvclass">)
          n3992 = local read "Accumulations"() -> (w4781:dbl)
          n3993 = call "LFA_Capture.vi"("error in (no error)"=w4784, "Frames"=w4781, "LightField Automation in"=w4785) -> ("error out"=w4783:errorcluster, "Data"=w4786:T26, "LightField Automation out"=w4782:refnum<class "LightField Automation.lvclass">)  [unwired: 6 in]
          n3994 = local write "LightField Automation out"(w4782) -> ()
          n3995 = local write "LightField Automation error out"(w4783) -> ()
        }
      }
      n3996 = local read "Acq Mode"() -> (w4738:T3)
      n3997 = case shown="\"Spectrum\", Default" w4738 {
        selector: w4738 -> [w4740 w4758]
        tunnel: w4739 -> [w4741 w4759]
        frame "Spectrum", Default {
          n3998 = stacked-sequence {
            tunnel: w4741 -> [_ w4752 _ _]
            tunnel: w4740 -> [_ w4750 _ _]
            frame #0 {
              n3999 = property on="CCD 2D Image Main" class="IntGraph (strict)"("Visible"=FALSE) -> ()  [unwired: 2 in, 2 out]
              n4000 = property on="CCD 1D Spectrum Main" class="XYGraph (strict)"("Visible"=TRUE) -> ()  [unwired: 2 in, 2 out]
            }
            frame #1 {
              n4001 = local read "Wavelength calibration"() -> (w4749:dbl[])
              n4002 = local read "CCD ROI"() -> (w4745:T20)
              n4003 = Divide(x=1239.842, y=w4749) -> (x/y=w4747:dbl[])
              n4004 = call "PrepareData4Graph.vi"("Wavelength nm"=w4747, "DataLF"=w4752, "CCD ROI"=w4745, "AcqMode"=w4750, "Data type"=T30."Spectre") -> ("Spectrum"=w4751:cluster{"Array 2":dbl[], "Array":dbl[]}, "PLInt out"=w4744:dbl[])  [unwired: 2 in, 2 out]
              n4005 = local write "CCD 1D Spectrum Main"(w4751) -> ()
              n4006 = local write "BackgroundSpec"(w4744) -> ()
            }
            frame #2 {
              n4007 = local read "BackgroundSpec"() -> (w4753:dbl[])
              n4008 = call-poly <vilib>:"Mean.vi"("X"=w4753) -> ("mean"=w4755:dbl)  [unwired: 1 out]
              n4009 = Negate(x=w4755) -> (-x=w4754:dbl)
              n4010 = property on="CCD 1D Spectrum Main" class="XYGraph (strict)"("YScale.Offset"=w4754) -> ()  [unwired: 2 in, 2 out]
            }
            frame #3 {
              n4011 = local write "Background taken?"(TRUE ("Background taken?")) -> ()
              n4012 = property on="Background substract" class="Enum (strict)"("Value"=enum16{"None", "Shutter"}."None" ("Background substract")) -> ()  [unwired: 2 in, 2 out]
            }
          }
        }
        frame "Image" {
          n4013 = stacked-sequence {
            tunnel: w4759 -> [_ w4767]
            tunnel: w4758 -> [_ w4765]
            frame #0 {
              n4014 = property on="CCD 2D Image Main" class="IntGraph (strict)"("Visible"=TRUE) -> ()  [unwired: 2 in, 2 out]
              n4015 = property on="CCD 1D Spectrum Main" class="XYGraph (strict)"("Visible"=FALSE) -> ()  [unwired: 2 in, 2 out]
            }
            frame #1 {
              n4016 = local read "Wavelength calibration"() -> (w4766:dbl[])
              n4017 = local read "CCD ROI"() -> (w4762:T20)
              n4018 = call "PrepareData4Graph.vi"("Wavelength nm"=w4766, "DataLF"=w4767, "CCD ROI"=w4762, "AcqMode"=w4765, "Data type"=T30."Spectre") -> ("Intensity Graph"=w4764:dbl[][])  [unwired: 2 in, 3 out]
              n4019 = local write "CCD 2D Image Main"(w4764) -> ()
            }
          }
        }
      }
    }
    frame Enabled {
    }
  }
  n4020 = disable-structure shown="Enabled" {
    frame Disabled {
    }
    frame Enabled {
      w4788 = dbl[] []
      w4794 = TRUE ("Visible")
      # "Progress bars"
      # "XYZ objective piezos and shutter"
      # "connected through"
      # "XY Scanning measurements"
      # "Polarisation measurement"
      # "Spectrum Custom"
      # "Spectrum with APDs"
      # "Acquire controls"
      # "Save controls"
      # "CCD"
      # "MonochromatorS"
      # "Rotation stages PR50PP"
      # "Main"
      # "Photodiode PM16-120"
      # "Steering mirror FSM 300"
      # "Settings for instrumentation"
      # "Contrôle manip GH013"
      n4021 = property on="CCD 1D Spectrum Main Energy Scale" class="XYGraph (strict)"("Plot.Visible?"=FALSE ("Plot.Visible"), "Plot.Line Width"=u8 0) -> ()  [unwired: 2 in, 2 out]
      n4022 = local write "Photodiode Status"(FALSE) -> ()
      n4023 = property on="Polarisation 1D Spectrum Energy Scale" class="XYGraph (strict)"("Plot.Visible?"=FALSE ("Plot.Visible"), "Plot.Line Width"=u8 0) -> ()  [unwired: 2 in, 2 out]
      n4024 = Bundle(w4788, w4788) -> (w4787:cluster{dbl[], dbl[]})  [unwired: 1 in]
      n4025 = Build Array(w4787, w4787) -> ()  [unwired: 1 out]
      n4026 = control-ref of="Scanning Mode"() -> (w4834:refnum<vi>)
      n4027 = control-ref of="Scan Fast Axis"() -> (w4835:refnum<vi>)
      n4028 = control-ref of="Scan X Num. Pts"() -> (w4831:refnum<vi>)
      n4029 = control-ref of="Spectrum End Wavelength (nm)"() -> (w4802:refnum<vi>)
      n4030 = control-ref of="Spectrum Step Wavelength (nm)"() -> (w4801:refnum<vi>)
      n4031 = control-ref of="Spectrum Start Wavelength (nm)"() -> (w4800:refnum<vi>)
      n4032 = control-ref of="Spectrum Custom Mode"() -> (w4799:refnum<vi>)
      n4033 = control-ref of="Scan Y Center (V)"() -> (w4830:refnum<vi>)
      n4034 = control-ref of="Scan X Center (V)"() -> (w4833:refnum<vi>)
      n4035 = control-ref of="Scan Y Tot. Length"() -> (w4796:refnum<vi>)
      n4036 = control-ref of="Scan Y Res. (V)"() -> (w4829:refnum<vi>)
      n4037 = control-ref of="Scan X Tot. Length (V)"() -> (w4797:refnum<vi>)
      n4038 = control-ref of="Scan Y Num. Pts"() -> (w4828:refnum<vi>)
      n4039 = property on="StopPolar" class="Bool (strict)"("Visible"=w4794) -> ()  [unwired: 2 in, 2 out]
      n4040 = property on="PausePolar" class="Bool (strict)"("Visible"=w4794) -> ()  [unwired: 2 in, 2 out]
      n4041 = control-ref of="Scan X Res. (V)"() -> (w4832:refnum<vi>)
      n4042 = control-ref of="Polar Start Angle (°)"() -> (w4826:refnum<vi>)
      n4043 = control-ref of="Polar Step Angle (°)"() -> (w4824:refnum<vi>)
      n4044 = control-ref of="Polar End Angle (°)"() -> (w4825:refnum<vi>)
      n4045 = Build Array(w4802, w4801, w4800, w4799) -> (→"Scan Spectrum Cust Params":refnum<vi>[])
      n4046 = Build Array(w4835, w4834, w4833, w4832, w4831, w4830, w4829, w4828, w4797, w4796) -> (→"Scan XY Map Params":refnum<vi>[])
      n4047 = control-ref of="Save Polarisation"() -> (w4791:refnum<vi>)
      n4048 = control-ref of="Acquire Polarisation"() -> (w4792:refnum<vi>)
      n4049 = control-ref of="Polar mode"() -> (w4823:refnum<vi>)
      n4050 = Build Array(w4823, w4826, w4825, w4824) -> (w4793:refnum<vi>[])
      "Scan Polar Params" <- w4793
      n4051 = Build Array (concatenate)(w4793, w4792, w4791) -> (→"Scan Polar AllParams":refnum<vi>[])
      n4052 = control-ref of="LinTFine Start Pos (usteps)"() -> (w4820:refnum<vi>)
      n4053 = control-ref of="LinTFines Step Pos (usteps)"() -> (w4819:refnum<vi>)
      n4054 = control-ref of="LinTFine End Pos (usteps)"() -> (w4818:refnum<vi>)
      n4055 = control-ref of="Acquire Contrast"() -> (w4809:refnum<vi>)
      n4056 = control-ref of="Save Michelson"() -> (w4804:refnum<vi>)
      n4057 = control-ref of="Acquire Michelson"() -> (w4805:refnum<vi>)
      n4058 = control-ref of="LinT Step Pos (mm)"() -> (w4807:refnum<vi>)
      n4059 = control-ref of="LinT Start Pos (mm)"() -> (w4808:refnum<vi>)
      n4060 = control-ref of="LinT End pos (mm)"() -> (w4806:refnum<vi>)
      n4061 = control-ref of="Stop Contrast"() -> (w4822:refnum<vi>)
      n4062 = control-ref of="Pause Contrast"() -> (w4821:refnum<vi>)
      n4063 = Build Array(w4808, w4807, w4806, w4820, w4819, w4818) -> (→"Scan Contrast Ctrls":refnum<vi>[])
      n4064 = Bundle("LinTFine Start Pos (usteps)"=w4820, "LinTFines Step Pos (usteps)"=w4819, "LinTFine End Pos (usteps)"=w4818, "Acquire Contrast"=w4809, "Stop Contrast"=w4822, "Pause Contrast"=w4821) -> ()  [unwired: 1 in, 1 out]
      n4065 = control-ref of="Scan Contrast Ctrls"() -> ()  [unwired: 1 out]
      n4066 = Bundle("LinT Start Pos (mm)"="LinT Start Pos (mm)", "LinT Step Pos (mm)"="LinT Step Pos (mm)", "LinT End pos (mm)"="LinT End pos (mm)", "LinTFine Start Pos (usteps)"="LinTFine Start Pos (usteps)", "LinTFines Step Pos (usteps)"="LinTFines Step Pos (usteps)", "LinTFine End Pos (usteps)"="LinTFine End Pos (usteps)") -> (→"Scan Translation Params":T27)  [unwired: 1 in]
      n4067 = Build Array(w4808, w4807, w4806, w4805, w4804) -> (→"Scan Translation Coarse Ctrls":refnum<vi>[])
      "ESP300 COM Port" <- refnum<visa-resource-name> "COM4" ("ESP300 COM Port")
      "PD 1D Spectrum" <- dbl[][] []
    }
  }
  n4068 = local write "DotNum"(0.0 ("DotNum")) -> ()
  n4069 = property on="Elapsed (s)" class="DigNum (strict)"("Visible"=w19) -> ()  [unwired: 2 in, 2 out]
  n4070 = disable-structure shown="Disabled" {
    disable-tunnel: w19 -> [w4841 _]
    frame Disabled {
      n4071 = property on="Scan Main Progess Bar" class="Slide (strict)"("Visible"=w4841) -> ()  [unwired: 2 in, 2 out]
    }
    frame Enabled {
    }
  }
  n4072 = property on="Acquire XY Map" class="Bool (strict)"("Visible"=w18, "Value"=FALSE ("Acquire XY Map")) -> ()  [unwired: 2 in, 2 out]
  n4073 = property on="Save XY Map" class="Bool (strict)"("Visible"=w18) -> ()  [unwired: 2 in, 2 out]
  n4074 = local write "Background taken?"(FALSE ("Background taken?")) -> ()
  n4075 = property on="Pause XY Map" class="Bool (strict)"("Visible"=w20, "Value"=w21) -> ()  [unwired: 2 in, 2 out]
  n4076 = property on="Stop XY Map" class="Bool (strict)"("Visible"=w20, "Value"=w21) -> ()  [unwired: 2 in, 2 out]
  n4077 = local write "BackgroundSpec"(i32[] []) -> ()
  n4078 = property on="Background substract" class="Enum (strict)"("Value"=enum16{"None", "Shutter"}."None" ("Background substract")) -> ()  [unwired: 2 in, 2 out]
  n4079 = control-ref of="Acquire Contrast"() -> (w9:refnum<vi>)
  n4080 = control-ref of="Save Contrast"() -> (w11:refnum<vi>)
  n4081 = property on="Save fPow" class="Bool (strict)"("Visible"=TRUE) -> ()  [unwired: 2 in, 2 out]
  n4082 = property class="Bool (strict)"(reference=w11, "DisabledEnum"=w10) -> ()  [unwired: 1 in, 2 out]
  n4083 = property on="Stop fPow" class="Bool (strict)"("Visible"=w16) -> ()  [unwired: 2 in, 2 out]
  n4084 = property on="Pause fPow" class="Bool (strict)"("Visible"=w16) -> ()  [unwired: 2 in, 2 out]
  n4085 = property class="Bool (strict)"(reference=w9, "DisabledEnum"=w10) -> ()  [unwired: 1 in, 2 out]
  n4086 = disable-structure shown="Enabled" {
    frame Enabled {
      # "Disabled because not coded (yet)"
    }
    frame Disabled {
    }
  }
  n4087 = control-ref of="MasterStop"() -> (w13:refnum<vi>)
  n4088 = control-ref of="MasterPause"() -> (w12:refnum<vi>)
  n4089 = property on="HR mode" class="Ring (strict)"("DisabledEnum"=T28."Enabled" ("Disabled")) -> ()  [unwired: 2 in, 2 out]
  n4090 = control-ref of="ExperimentStopped?"() -> (w14:refnum<vi>)
  n4091 = call "CheckStopAndReset.vi"("ExperimentStopped?"=w14, "MasterStop"=w13, "MasterPause"=w12) -> ()
  n4092 = control-ref of="Mono2 Wavelength (nm)"() -> ()  [unwired: 1 out]
  n4093 = control-ref of="Save PLE"() -> (w4:refnum<vi>)
  n4094 = control-ref of="PLE Start (nm)"() -> (w8:refnum<vi>)
  n4095 = control-ref of="PLE End (nm)"() -> (w7:refnum<vi>)
  n4096 = control-ref of="PLE Step (nm)"() -> (w6:refnum<vi>)
  n4097 = control-ref of="Acquire PLE"() -> (w5:refnum<vi>)
  n4098 = control-ref of="MasterStop"() -> ()  [unwired: 1 out]
  n4099 = control-ref of="MasterPause"() -> ()  [unwired: 1 out]
  n4100 = Build Array(w5, w4, w8, w7, w6) -> (→"Scan PLE AllParams":refnum<vi>[])
  n4101 = control-ref of="Pause fPow"() -> ()  [unwired: 1 out]
  n4102 = property on="Elapsed (s)" class="DigNum (strict)"("Visible"=FALSE) -> ()  [unwired: 2 in, 2 out]
  n4103 = disable-structure shown="Enabled" {
    frame Enabled {
      # "Documentation Buttons"
    }
    frame Disabled {
    }
  }
  n4104 = property on="HR mode" class="Ring (strict)"("DisabledEnum"=T28."Disabled and Grayed Out" ("Disabled")) -> ()  [unwired: 2 in, 2 out]
  "Background taken?" <- FALSE ("Background taken?")
